vi "transceiverRFID v3 queue.vi"() -> ()   [LabVIEW 2015]
uses:
  <instrlib>/niUSRP/niUSRP Write Tx Data (CDB).vi
  <instrlib>/niUSRP/niUSRP Fetch Rx Data (CDB Cluster).vi
  <vilib>/measure/mamon.llb/Trigger Detection for 1 Channel.vi
  <vilib>/Waveform/WDTOps.llb/WDT Get Waveform Subset DBL.vi
  <vilib>/measure/NI_MAPro.lvlib
panel:
  out "Tx stop?":bool
  out "error out 3":errorcluster
  in  "Parameters Query":T1 {"Session" items=["S0", "S1", "S2", "S3"]; "Sel" items=["All", "All2", "~SL", "SL"]; "M" items=["M=1", "M=2", "M=4", "M=8"]}
  in  "Symbol Rate [Hz]":dbl=500000.0 format="%#_13p"
  in  "Parameters Select":T2={"Target"=7, "Action"=0, "MemBank"=1, "truncate"=FALSE} {"MemBank" items=["00 RFU", "01 EPC", "10 TID", "11 User"]; "Action" items=["000", "001", "010", "011", "100", "101", "110", "111"]; "Target" items=["000 Inventoried (S0)", "001 Inventoried (S1)", "010 Inventoried (S2)", "011 Inventoried (S3)", "100 SL", "101 RFU", "110 RFU", "111 RFU"]}
  in  "Parameters Symbols":T3={"Tari"=8e-06, "PW"=0.5, "factor for \"1\" symbol"=0.5, "RTcal"=2.5, "TRcal"=3.0, "Delimiter"=1.4e-05} {"TRcal" min=1.1 max=3.0 step=0.1; "RTcal" min=2.5 max=3.0 step=0.1; "factor for \"1\" symbol" min=0.5 max=1.0 step=0.1; "PW" min=0.265 max=0.525 step=0.001; "Tari" format="%#_3p"}
  out "coerced IQ rate 2":dbl=100000.0 format="%#_6p"
  out "carrier frequency 3":dbl=100000.0 format="%#_6p"
  out "coerced gain 2":dbl format="%#_6f"
  in  "stop":bool
  out "Rx Loop":i32
  out "RFID Pushed":bool
  in  "query":bool
  out "RN16 array":i32[](array[numeric])=[0, 1, 1, 0, 0, 0, 1, 0, 1, 1, 1, 1, 1, 1, 1, 1]
  out "bits":i16[](graph)=[1, 1, 1, 1, 0, 0, 1, 0, 0, 0, 1, 1, 0, 0, 0, 0, 0, 1, 1, 1, 0, 0, 1, 0, 0, 0, 0, 1, 1, 1, 0, 0, 1, 0, 0, 1, 0, 0, 1, 0, 0, 0, 0, 1, 1, 0, 1, 1, 1, 0, 0, 0, 0, 1, 1, 1, 0, 0, 0, 1, 1, 1, 0, 0, 0, 0, 1, 1, 1, 0, 0, 0, 0, 1, 1, 1, 0, 0, 0, 0, 0, 0, 0, 0]
  out "Wave Mag":dbl[](graph)
  out "ACK":bool
  in  "IQ rate 2":dbl=2000000.0 format="%#_6p"
  in  "carrier frequency 2":dbl=920000000.0 format="%#_6p"
  in  "gain 2":dbl format="%#_6f"
  in  "tx device names":refnum<k15>="192.168.20.13"
  in  "active antenna":string="RX2"
  in  "Channels":string(combo)="0"
  in  "timeout":dbl=10.0
  in  "number of samples":i64=2000000
  in  "Stop":bool
  out "Magnitude":cluster{"t0":dbl, "dt":dbl, "Y":dbl[]}(graph)={"t0"=425.94010384, "dt"=5e-07, "Y"=array[2000000 elements]}
  out "Triggered Signal":dynamicdata(graph)=[{"t0"=timestamp(16448802 s since 1904-01-01), "dt"=1.0, "Y"=array[750 elements], "attributes"=variant("NI_ChannelName"=variant(string "Trigger"))}]
  out "Portion Signal":dynamicdata(graph)=[{"t0"=timestamp(3606796793.4692063 s since 1904-01-01), "dt"=1.0, "Y"=[0.175, 0.175, 0.175, 0.175, 0.215, 0.215, 0.215, 0.175, 0.175, 0.215, 0.215, 0.175, 0.175, 0.175, 0.215, 0.215, 0.175, 0.215, 0.215, 0.175, 0.175, 0.215, 0.175, 0.175, 0.215, 0.215, 0.175, 0.215, 0.215, 0.175, 0.175, 0.215, 0.175, 0.175, 0.215, 0.175, 0.175, 0.215, 0.215, 0.175, 0.215, 0.215, 0.175, 0.175, 0.215, 0.175, 0.175, 0.215, 0.175, 0.175, 0.215, 0.215, 0.175, 0.175, 0.215, 0.175, 0.175, 0.215, 0.175, 0.175, 0.215, 0.215, 0.215, 0.175, 0.175, 0.215, 0.175, 0.175, 0.175, 0.175, 0.215, 0.215, 0.215, 0.175, 0.175, 0.215, 0.175, 0.175, 0.215, 0.175, 0.175, 0.215, 0.215, 0.175, 0.175, 0.215, 0.175, 0.175, 0.215, 0.175, 0.175, 0.215, 0.175, 0.175, 0.215, 0.215, 0.175, 0.175, 0.215, 0.175, 0.175, 0.215, 0.175, 0.175, 0.215, 0.215, 0.175, 0.175, 0.215, 0.175, 0.175, 0.215, 0.175, 0.175, 0.215, 0.215, 0.175, 0.215, 0.215, 0.175, 0.175, 0.215, 0.175, 0.175, 0.215, 0.175, 0.175, 0.215, 0.215, 0.175, 0.175, 0.215, 0.175, 0.175, 0.215, 0.175, 0.175, 0.215, 0.175, 0.175, 0.215, 0.215, 0.175, 0.175, 0.215, 0.175, 0.175, 0.215, 0.175, 0.175, 0.215, 0.215, 0.175, 0.175, 0.215, 0.175, 0.175, 0.215, 0.175, 0.175, 0.215, 0.175, 0.175, 0.215, 0.215, 0.175, 0.175, 0.215, 0.175, 0.175, 0.215, 0.175, 0.175, 0.215, 0.175, 0.175, 0.215, 0.215, 0.175, 0.175]}, {"t0"=timestamp(16449352 s since 1904-01-01), "dt"=1.0, "Y"=[0.6542204406555878, 0.6330066792866885, 0.6289206010452267, 0.626525788591559, 0.6440170826344898, 0.6558913247662658, 0.6551466050382949, 0.6446576873057327, 0.6276789703693967, 0.6487660336682352, 0.6515045603831945, 0.6315654455000962, 0.6285598365750038, 0.6291977552419075, 0.6513744582179881, 0.6487718708937794, 0.6281161281271066, 0.6441036383531251, 0.6540546398928915, 0.6323048994250363, 0.6359679052689398, 0.6558585780757112, 0.6396687990551979, 0.629156140414305, 0.6518867729873677, 0.6483523017326835, 0.6287998621524823, 0.6479419819057154, 0.6523620464006552, 0.6302348513521957, 0.6394592548080206, 0.6560056754287461, 0.6353038672852097, 0.6346389862773866, 0.6557564358134849, 0.6402277966255374, 0.6287483168841594, 0.651006297610194, 0.6487867644817977, 0.6294605495842085, 0.6476222426699878, 0.652197032759818, 0.6297422152107712, 0.638725861964971, 0.6556999088508416, 0.6357702096227417, 0.6303899874831843, 0.6536513023112432, 0.6453874681954346, 0.6282678144317502, 0.6470302178597716, 0.6522701409900283, 0.6299221874750973, 0.642426414545514, 0.6547052180570018, 0.6323249481039205, 0.6333552552398422, 0.6553467581989884, 0.6405086905627353, 0.6315662027705019, 0.6526133380528634, 0.6535557019281786, 0.654421911761707, 0.6380373636097645, 0.6307874460100164, 0.6536176318748712, 0.6406224634572578, 0.6270835009019179, 0.6269903627063104, 0.6338698329632815, 0.6536116384280213, 0.653257077985277, 0.6533937223519337, 0.6338942026134534, 0.6331043491528318, 0.6547473769267388, 0.6411190331089638, 0.6275601609203197, 0.6496280391371777, 0.6458061649598519, 0.6267659422503373, 0.6452588001110147, 0.6524795072180846, 0.6299948003589266, 0.6366571347752407, 0.6536005142113043, 0.632409054009175, 0.6318732943523131, 0.6539270504909295, 0.6414501140307582, 0.6276388315395326, 0.6491703842752117, 0.6458834206984477, 0.6262937266147462, 0.6443153980416729, 0.6519924520978075, 0.629042357653491, 0.6353287837179523, 0.6545296689316882, 0.6369081613804035, 0.6290638058284929, 0.6512822332544489, 0.6457777456866854, 0.6263645066376707, 0.6442292350994769, 0.6496124314718684, 0.6268011308873612, 0.6393831799145786, 0.6540143802735646, 0.633088873311549, 0.6314470575578446, 0.6529060917394062, 0.6369507583109556, 0.6280382313641445, 0.6507502705684688, 0.6457390376488532, 0.6257248776510101, 0.6436289616350072, 0.6499581940450706, 0.6274609957119216, 0.6388504902100247, 0.6536636816864714, 0.6331735786644757, 0.6306605221497352, 0.652740208254182, 0.64128117204542, 0.6258860788907208, 0.6468182432467872, 0.6496205615265724, 0.6272331501727273, 0.6382326153017709, 0.6518270541144702, 0.629643965384008, 0.6335678245703787, 0.6533675162201217, 0.6366936469982558, 0.6262540961233908, 0.6495447267673374, 0.6419769674391187, 0.6253642504421832, 0.6456429465893609, 0.6490760180330309, 0.6268146564515095, 0.6374754890127863, 0.6517341322079381, 0.6289016397242593, 0.6323826159966556, 0.6531167564613976, 0.637130944131767, 0.626625252663772, 0.6488663115123084, 0.6458866479589179, 0.6257091686813125, 0.6408464802006677, 0.6515973320665904, 0.628676080037199, 0.6319590623959827, 0.652097765579169, 0.633324553683118, 0.6285426588530133, 0.6505853921308588, 0.6415519048673486, 0.6245075306846388, 0.6447252096283556, 0.6459387707408372, 0.6241539664908139, 0.6401210700943205, 0.6516950719440161, 0.6296678507097518, 0.6316662953086386, 0.6517458063157089, 0.6333743530720075, 0.627704200597501, 0.6504285603489174, 0.6412976730640289, 0.6238942612116077, 0.6437532229968528, 0.649057237990462, 0.6263972072140956, 0.6345010038828095], "attributes"=variant("NI_ChannelName"=variant(string "Trigger"))}]
  out "start samples":dbl format="%.3g"
  out "duration samples":dbl format="%.3g"
  in  "start":i64=550 format="%.3g"
  in  "duration":dbl=180.0 format="%#_13g"
  out "RN16 waveform":i16[](graph)
  out "error out 2":errorcluster
  out "Tx loop":i32
  out "trigger location":dbl format="%#_2g"
  out "Trigger":bool
  out "coerced gain":dbl format="%#_6f"
  out "coerced carrier frequency":dbl=100000.0 format="%#_6p"
  out "coerced IQ rate":dbl=100000.0 format="%#_6p"
  in  "gain":dbl format="%#_6f"
  in  "carrier frequency":dbl=920000000.0 format="%#_6p"
  in  "IQ rate":dbl=2000000.0 format="%#_6p"
  out "error out":errorcluster
  in  "device names":refnum<k15>="192.168.10.14"
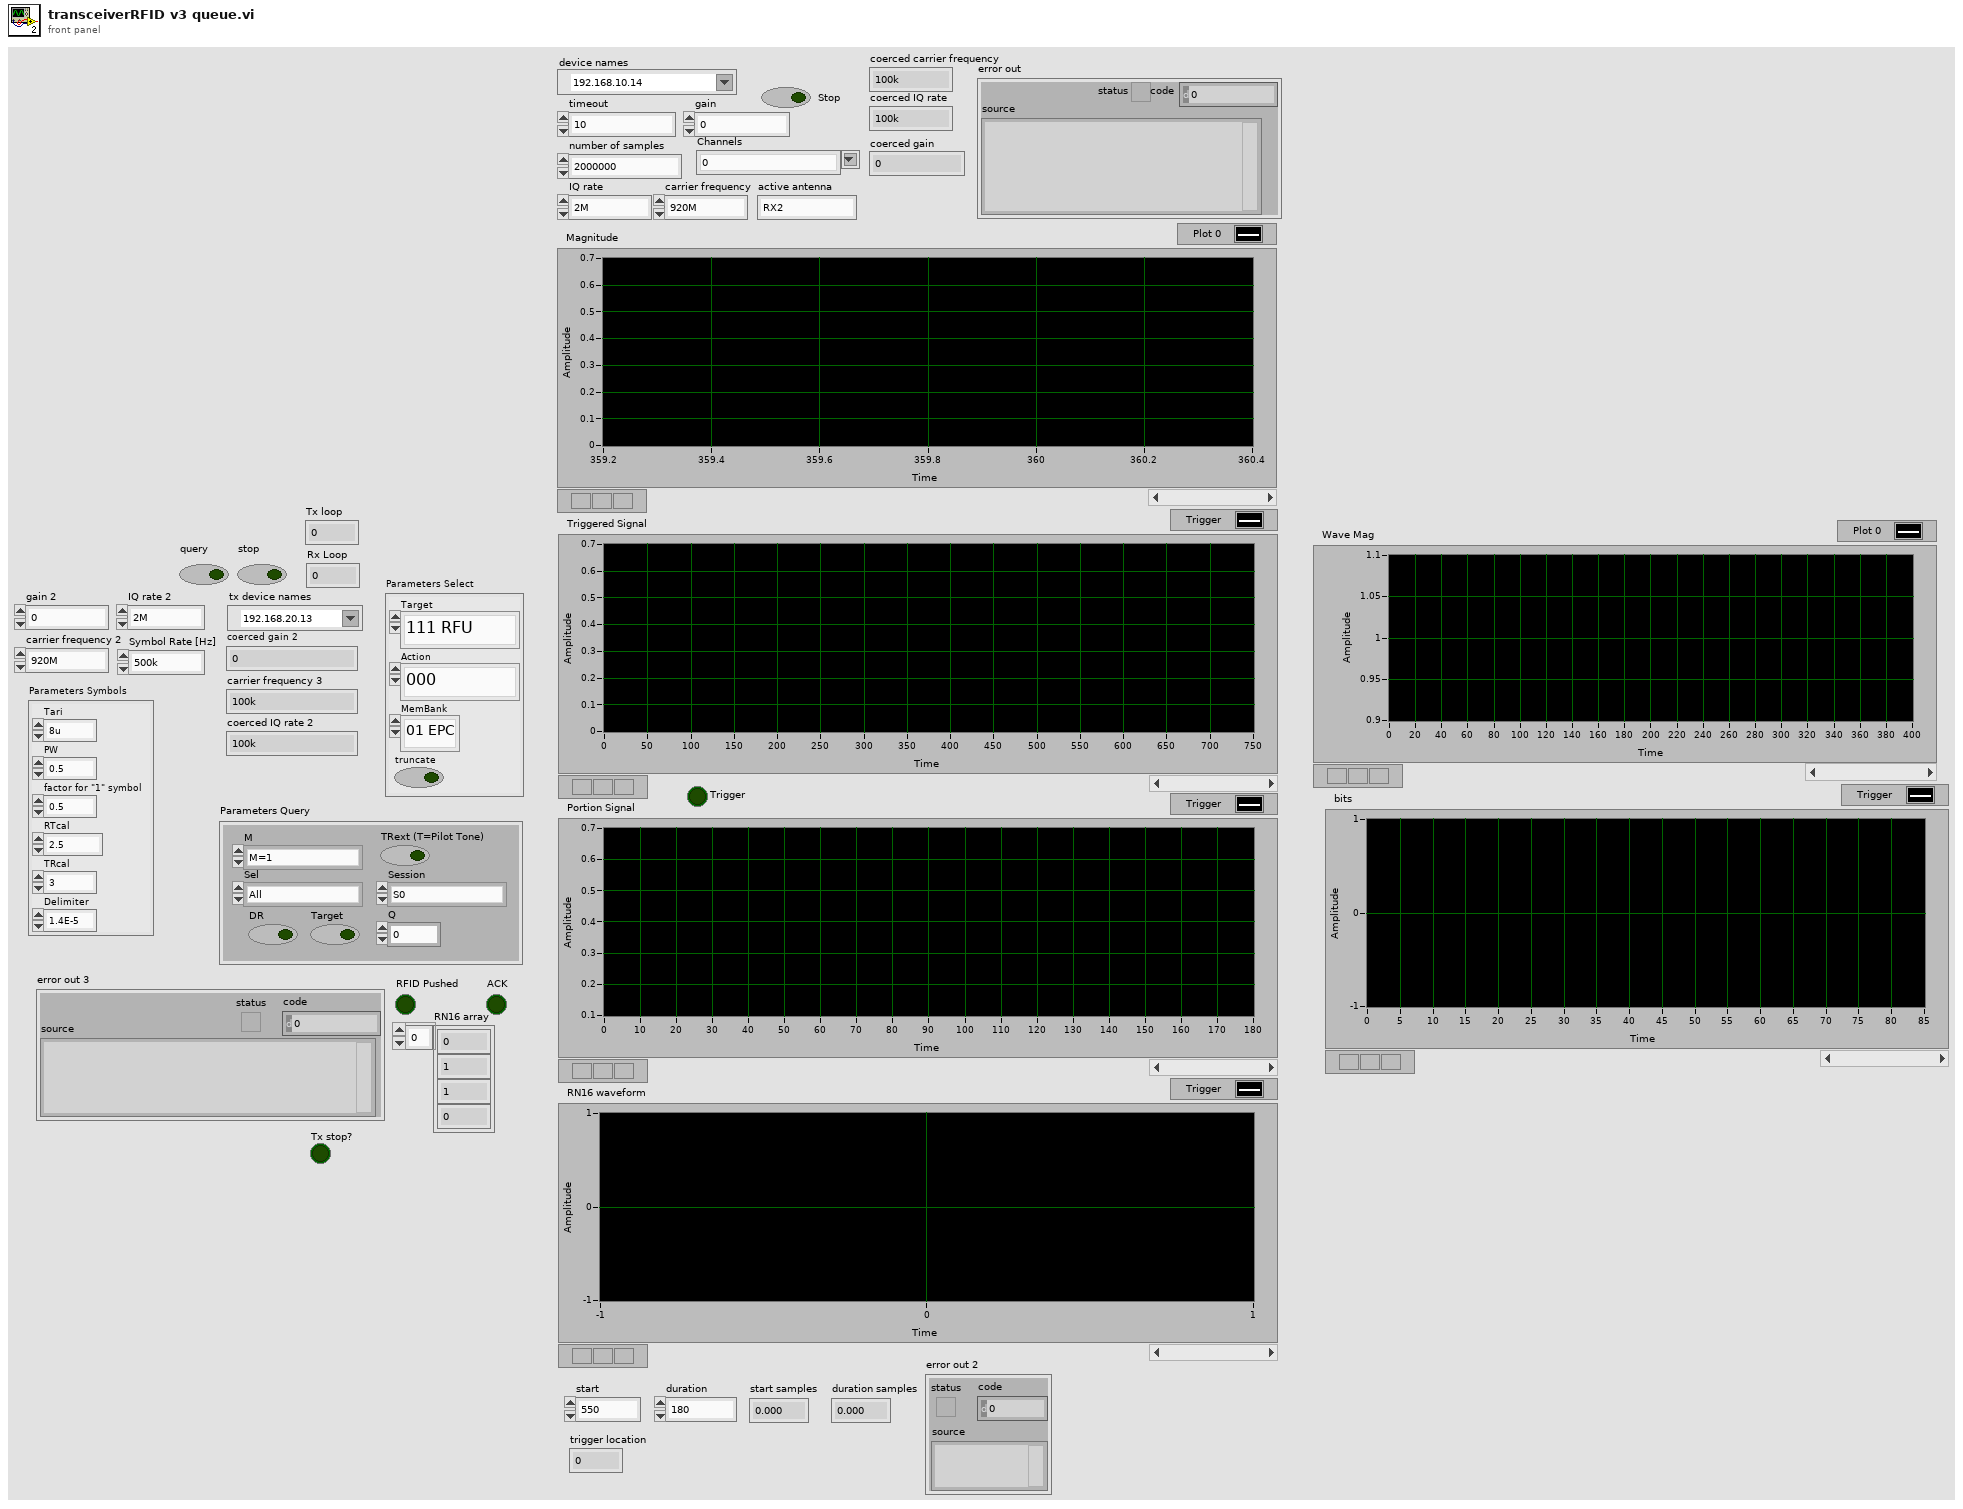
[diagram p1: front panel]
types:
  T1 = cluster{"DR":bool, "M":u16, "TRext (T=Pilot Tone)":bool, "Sel":u16, "Session":u16, "Q":u8, "Target":bool}
  T2 = cluster{"Target":u16, "Action":u16, "MemBank":u16, "truncate":bool}
  T3 = cluster{"Tari":dbl, "PW":dbl, "factor for \"1\" symbol":dbl, "RTcal":dbl, "TRcal":dbl, "Delimiter":dbl}
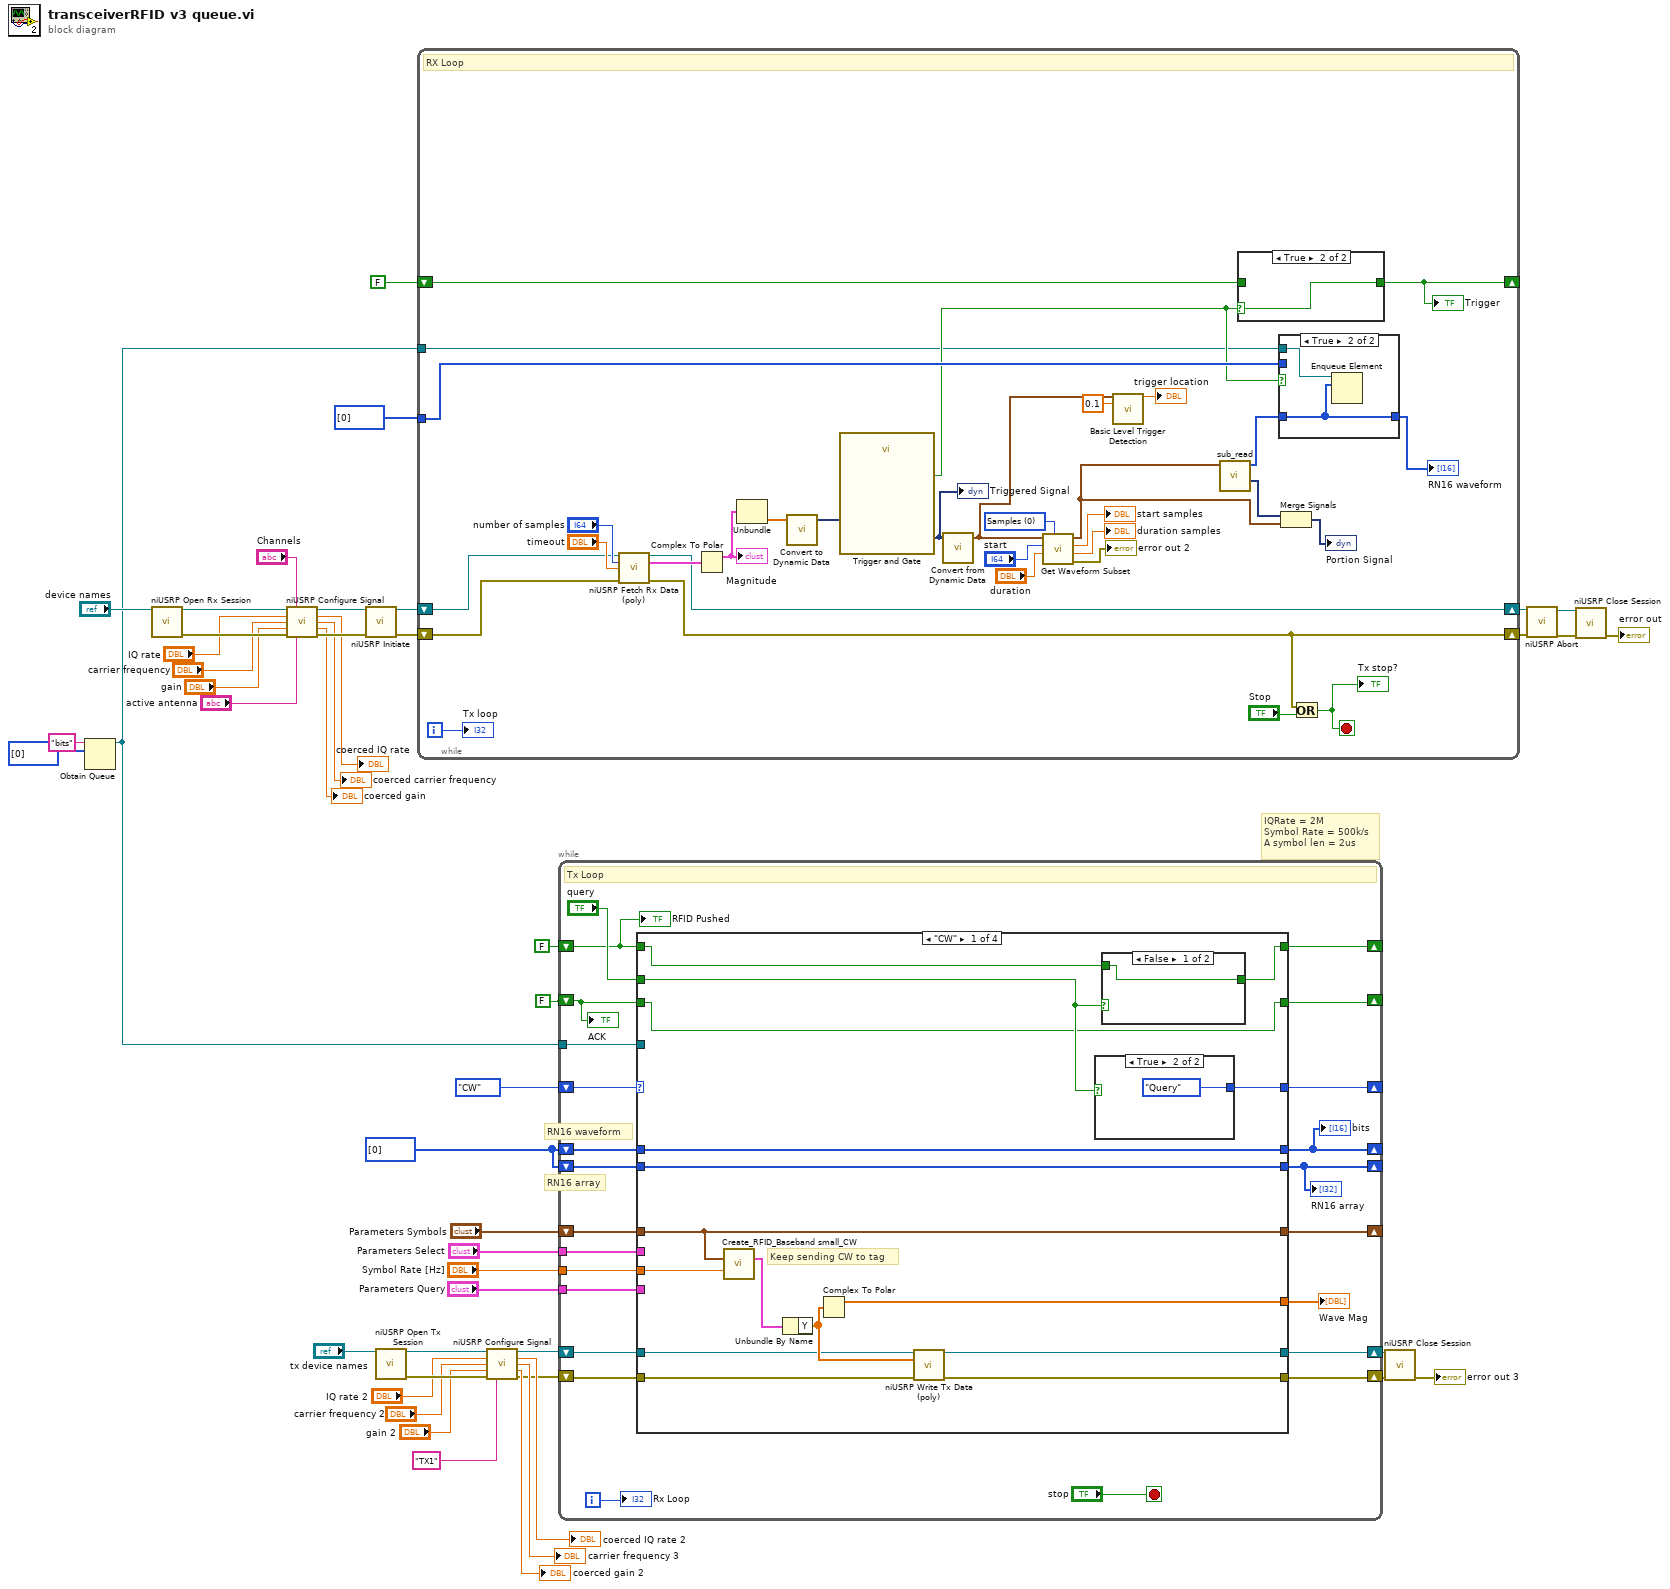
[diagram p0: block diagram]
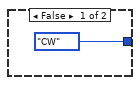
[diagram p3: hidden frame]
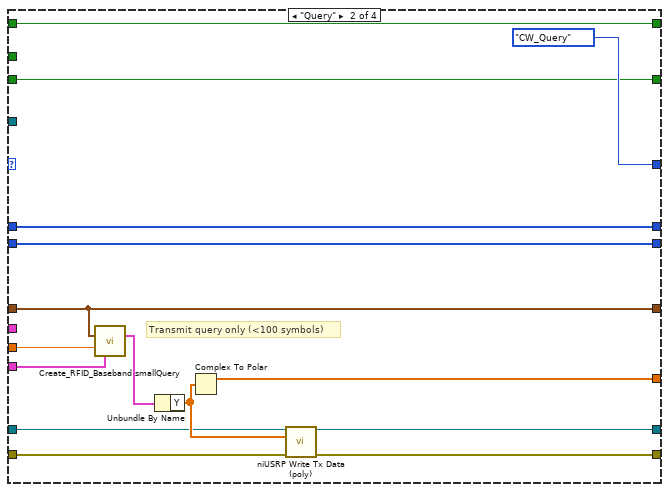
[diagram p4: hidden frame]
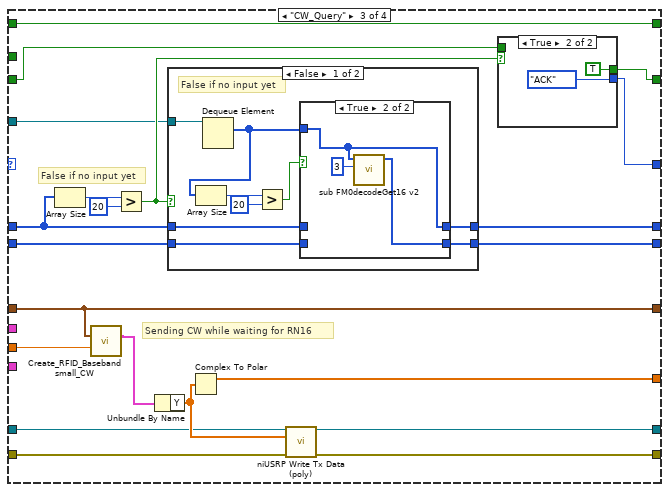
[diagram p5: hidden frame]
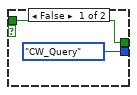
[diagram p6: hidden frame]
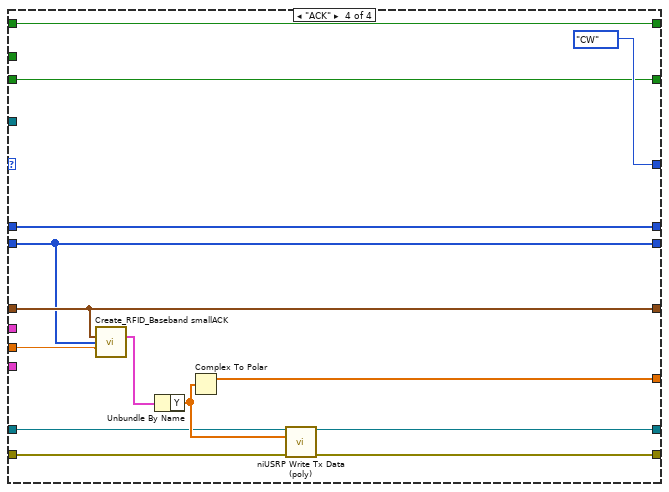
[diagram p9: hidden frame]
diagram:
  w5 = i16[] [0]
  # "IQRate = 2M\nSymbol Rate = 500k/s\nA symbol len = 2us"
  # "RN16 array"
  # "RN16 waveform"
  n1 = Obtain Queue(name (unnamed)="bits", element data type=i16[] [0]) -> (queue out=w2:refnum<queue>)  [unwired: 3 in, 2 out]
  n2 = call <instrlib>:"niUSRP Open Rx Session.vi"("device names"="device names") -> ("session handle out"=w47:refnum<k15>, "error out"=w46:errorcluster)  [unwired: 13 in]
  n3 = call <instrlib>:"niUSRP Configure Signal.vi"("session handle"=w47, "channel list"="Channels", "IQ rate"="IQ rate", "carrier frequency"="carrier frequency", "gain"="gain", "error in (no error)"=w46, "active antenna"="active antenna") -> ("session handle out"=w45:refnum<k15>, "coerced IQ rate"=→"coerced IQ rate":dbl, "coerced carrier frequency"=→"coerced carrier frequency":dbl, "coerced gain"=→"coerced gain":dbl, "error out"=w44:errorcluster)  [unwired: 4 in]
  n4 = call <instrlib>:"niUSRP Initiate.vi"("session handle"=w45, "error in (no error)"=w44) -> ("session handle out"=w43:refnum<k15>, "error out"=w42:errorcluster)  [unwired: 12 in]
  n5 = call <instrlib>:"niUSRP Open Tx Session.vi"("device names"="tx device names") -> ("session handle out"=w8:refnum<k15>, "error out"=w26:errorcluster)  [unwired: 13 in]
  n6 = while {
    shift-right: [w78] -> w41
    shift-left: w43 -> [w77]
    shift-right: [w61] -> w40
    shift-left: w42 -> [w76]
    shift-right: [w54] -> _
    shift-left: FALSE -> [w53]
    tunnel: i16[] [0] -> [w58]
    tunnel: w2 -> [w49]
    i -> [w60]
    stop <- w73 stop-if-true
    w70 = u16 0 items=["Samples", "Relative Time"] ("start/duration format")
    # "RX Loop"
    n7 = call-poly <instrlib>:"niUSRP Fetch Rx Data (poly).vi"("session handle"=w77, "number of samples"="number of samples", "timeout"="timeout", "error in (no error)"=w76) -> ("session handle out"=w78:refnum<k15>, "data"=w79:cluster{"t0":dbl, "dt":dbl, "Y":cdb[]}, "error out"=w61:errorcluster)  [unwired: 8 in, 1 out]
    n8 = Complex To Polar(r * e^(i*theta)=w79) -> (r=w75:cluster{"t0":dbl, "dt":dbl, "Y":dbl[]})  [unwired: 1 out]
    "Magnitude" <- w75
    n9 = Unbundle(w75) -> ("Y"=w64:dbl[])  [unwired: 2 out]
    n10 = call "Convert to Dynamic Data"("Array"=w64) -> ("Dynamic Data Type"=w74:dynamicdata)  [unwired: 3 in]
    n11 = call "Trigger and Gate"("Signals"=w74) -> ("Triggered Signals"=w67:dynamicdata, "Data Available"=w52:bool)  [unwired: 7 in, 2 out]
    "Triggered Signal" <- w67
    n12 = call "Convert from Dynamic Data"("Dynamic Data Type"=w67) -> ("Waveform"=w55:waveform(dbl))  [unwired: 3 in]
    n13 = call-poly <vilib>:"Get Waveform Subset.vi"("start/duration format"=w70, "duration"="duration", "start samples/time"="start", "waveform in"=w55) -> ("error out"=→"error out 2":errorcluster, "actual duration"=→"duration samples":dbl, "actual start samples/time"=→"start samples":dbl, "waveform out"=w57:waveform(dbl))  [unwired: 2 in]
    n14 = call-poly <vilib>:"Basic Level Trigger Detection.vi"("signal in"=w55, "level"=0.1) -> ("trigger location"=→"trigger location":dbl)  [unwired: 11 in, 2 out]
    n15 = call "sub_read.vi"("Raw Signal"=w57) -> ("Digitized Sign"=w66:dynamicdata, "Bits"=w59:i16[])  [unwired: 6 in, 2 out]
    n16 = case shown="True" w52 {
      selector: w52 -> [_ w83]
      tunnel: [w82 w83] -> w54
      tunnel: w53 -> [w82 _]
      frame False {
      }
      frame True {
      }
    }
    "Trigger" <- w54
    n17 = case shown="True" w52 {
      tunnel: w59 -> [_ w86]
      tunnel: [w84 w86] -> w50
      tunnel: w58 -> [w84 _]
      tunnel: w49 -> [_ w85]
      frame False {
      }
      frame True {
        n18 = Enqueue Element(queue=w85, element=w86) -> ()  [unwired: 2 in, 3 out]
      }
    }
    "RN16 waveform" <- w50
    n19 = Merge Signals(w66, w57) -> (→"Portion Signal":dynamicdata)
    n20 = Or(x=w61, y="Stop") -> (x .or. y?=w73:bool)
    "Tx stop?" <- w73
    "Tx loop" <- w60
  }
  n21 = call <instrlib>:"niUSRP Configure Signal.vi"("session handle"=w8, "IQ rate"="IQ rate 2", "carrier frequency"="carrier frequency 2", "gain"="gain 2", "error in (no error)"=w26, "active antenna"="TX1") -> ("session handle out"=w1:refnum<k15>, "coerced IQ rate"=→"coerced IQ rate 2":dbl, "coerced carrier frequency"=→"carrier frequency 3":dbl, "coerced gain"=→"coerced gain 2":dbl, "error out"=w13:errorcluster)  [unwired: 5 in]
  n22 = while {
    tunnel: "Parameters Select" -> [w104]
    tunnel: "Parameters Query" -> [w102]
    shift-right: [w107] -> w12
    shift-left: w13 -> [w108]
    shift-right: [w106] -> w10
    shift-left: w1 -> [w87]
    shift-right: [w99] -> _
    shift-left: enum16{"CW", "Query", "CW_Query", "ACK"}."CW" -> [w109]
    shift-right: [w101] -> _
    shift-left: "Parameters Symbols" -> [w105]
    tunnel: "Symbol Rate [Hz]" -> [w103]
    shift-right: [w97] -> _
    shift-left: w5 -> [w98]
    shift-right: [w96] -> _
    shift-left: w5 -> [w95]
    shift-right: [w92] -> _
    shift-left: FALSE ("query") -> [w91]
    shift-right: [w89] -> _
    shift-left: FALSE ("query") -> [w90]
    tunnel: w2 -> [w88]
    i -> [w110]
    stop <- "stop" stop-if-true
    # "Tx Loop"
    n23 = case shown="\"CW\"" w109 {
      tunnel: w87 -> [w125 w144 w165 w199]
      tunnel: w108 -> [w124 w143 w164 w198]
      tunnel: [w123 w142 w163 w197] -> w107
      tunnel: [w122 w141 w162 w196] -> w106
      tunnel: w105 -> [w120 w136 w153 w194]
      tunnel: w104 -> [_ _ _ _]
      tunnel: w103 -> [w119 w137 w152 w193]
      tunnel: w102 -> [_ w138 _ _]
      tunnel: [w120 w136 w153 w194] -> w101
      tunnel: [w121 w140 w161 w195] -> w94
      tunnel: [w117 enum16{"CW", "Query", "CW_Query", "ACK"}."CW_Query" w150 enum16{"CW", "Query", "CW_Query", "ACK"}."CW"] -> w99
      tunnel: "query" -> [w114 _ _ _]
      tunnel: w98 -> [w116 w135 w158 w190]
      tunnel: [w116 w135 w156 w190] -> w97
      tunnel: [w115 w134 w157 w191] -> w96
      tunnel: w95 -> [w115 w134 w155 w191]
      tunnel: [w113 w132 w149 w188] -> w92
      tunnel: w91 -> [w112 w132 w149 w188]
      tunnel: w90 -> [w111 w131 w148 w187]
      tunnel: [w111 w131 w147 w187] -> w89
      tunnel: w88 -> [_ _ w146 _]
      frame "CW" {
        # "Keep sending CW to tag"
        n24 = call "Create_RFID_Baseband small_CW.vi"("Parameters Symbols"=w120, "Symbol Rate [Hz]"=w119) -> ("complex waveform"=w118:cluster{"t0":dbl, "dt":dbl, "Y":cdb[]})  [unwired: 12 in, 1 out]
        n25 = Unbundle By Name(w118) -> ("Y"=w126:cdb[])
        n26 = Complex To Polar(r * e^(i*theta)=w126) -> (r=w121:dbl[])  [unwired: 1 out]
        n27 = call-poly <instrlib>:"niUSRP Write Tx Data (poly).vi"("session handle"=w125, "data"=w126, "error in (no error)"=w124) -> ("session handle out"=w122:refnum<k15>, "error out"=w123:errorcluster)  [unwired: 11 in]
        n28 = case shown="True" w114 {
          tunnel: [enum16{"CW", "Query", "CW_Query", "ACK"}."CW" enum16{"CW", "Query", "CW_Query", "ACK"}."Query"] -> w117
          frame False {
          }
          frame True {
          }
        }
        n29 = case shown="False" w114 {
          selector: w114 -> [_ w128]
          tunnel: [w127 w128] -> w113
          tunnel: w112 -> [w127 _]
          frame False {
          }
          frame True {
          }
        }
      }
      frame "Query" {
        # "Transmit query only (<100 symbols)"
        n30 = call "Create_RFID_Baseband smallQuery.vi"("Parameters Symbols"=w136, "Symbol Rate [Hz]"=w137, "Parameters Query"=w138) -> ("complex waveform"=w139:cluster{"t0":dbl, "dt":dbl, "Y":cdb[]})  [unwired: 11 in, 1 out]
        n31 = Unbundle By Name(w139) -> ("Y"=w145:cdb[])
        n32 = Complex To Polar(r * e^(i*theta)=w145) -> (r=w140:dbl[])  [unwired: 1 out]
        n33 = call-poly <instrlib>:"niUSRP Write Tx Data (poly).vi"("session handle"=w144, "data"=w145, "error in (no error)"=w143) -> ("session handle out"=w141:refnum<k15>, "error out"=w142:errorcluster)  [unwired: 11 in]
      }
      frame "CW_Query" {
        # "False if no input yet"
        # "Sending CW while waiting for RN16"
        n34 = Array Size(array=w158) -> (size(s)=w159:i32)
        n35 = call "Create_RFID_Baseband small_CW.vi"("Parameters Symbols"=w153, "Symbol Rate [Hz]"=w152) -> ("complex waveform"=w154:cluster{"t0":dbl, "dt":dbl, "Y":cdb[]})  [unwired: 12 in, 1 out]
        n36 = Greater?(x=w159, y=20) -> (0:w151:bool)
        n37 = Unbundle By Name(w154) -> ("Y"=w166:cdb[])
        n38 = case shown="False" w151 {
          tunnel: [w176 w186] -> w156
          tunnel: w158 -> [w173 w186]
          tunnel: [w175 w185] -> w157
          tunnel: w155 -> [w174 w185]
          tunnel: w146 -> [w172 _]
          frame False {
            # "False if no input yet"
            n39 = Dequeue Element(queue=w172) -> (element=w171:i16[])  [unwired: 2 in, 3 out]
            n40 = Array Size(array=w171) -> (size(s)=w179:i32)
            n41 = Greater?(x=w179, y=20) -> (0:w177:bool)
            n42 = case shown="True" w177 {
              tunnel: w173 -> [w181 _]
              tunnel: [w181 w182] -> w176
              tunnel: [w180 w184] -> w175
              tunnel: w174 -> [w180 _]
              tunnel: w171 -> [_ w182]
              frame False {
              }
              frame True {
                n43 = call "sub FM0decodeGet16 v2.vi"("threshold"=3, "RN16 waveform"=w182) -> ("RN16 array"=w184:i32[])  [unwired: 9 in]
              }
            }
          }
          frame True {
          }
        }
        n44 = Complex To Polar(r * e^(i*theta)=w166) -> (r=w161:dbl[])  [unwired: 1 out]
        n45 = call-poly <instrlib>:"niUSRP Write Tx Data (poly).vi"("session handle"=w165, "data"=w166, "error in (no error)"=w164) -> ("session handle out"=w162:refnum<k15>, "error out"=w163:errorcluster)  [unwired: 11 in]
        n46 = case shown="True" w151 {
          tunnel: [enum16{"CW", "Query", "CW_Query", "ACK"}."CW_Query" enum16{"CW", "Query", "CW_Query", "ACK"}."ACK"] -> w150
          tunnel: w148 -> [w167 _]
          tunnel: [w167 TRUE ("query")] -> w147
          frame False {
          }
          frame True {
          }
        }
      }
      frame "ACK" {
        n47 = call "Create_RFID_Baseband smallACK.vi"("Parameters Symbols"=w194, "RN16 array"=w191, "Symbol Rate [Hz]"=w193) -> ("complex waveform"=w192:cluster{"t0":dbl, "dt":dbl, "Y":cdb[]})  [unwired: 11 in, 1 out]
        n48 = Unbundle By Name(w192) -> ("Y"=w200:cdb[])
        n49 = Complex To Polar(r * e^(i*theta)=w200) -> (r=w195:dbl[])  [unwired: 1 out]
        n50 = call-poly <instrlib>:"niUSRP Write Tx Data (poly).vi"("session handle"=w199, "data"=w200, "error in (no error)"=w198) -> ("session handle out"=w196:refnum<k15>, "error out"=w197:errorcluster)  [unwired: 11 in]
      }
    }
    "RN16 array" <- w96
    "bits" <- w97
    "Wave Mag" <- w94
    "Rx Loop" <- w110
    "RFID Pushed" <- w91
    "ACK" <- w90
  }
  n51 = call <instrlib>:"niUSRP Close Session.vi"("session handle"=w10, "error in (no error)"=w12) -> ("error out"=→"error out 3":errorcluster)  [unwired: 13 in]
  n52 = call <instrlib>:"niUSRP Abort.vi"("session handle"=w41, "error in (no error)"=w40) -> ("session handle out"=w39:refnum<k15>, "error out"=w38:errorcluster)  [unwired: 12 in]
  n53 = call <instrlib>:"niUSRP Close Session.vi"("session handle"=w39, "error in (no error)"=w38) -> ("error out"=→"error out":errorcluster)  [unwired: 13 in]
